vi "ImageInputToMatrix.vi"(0 "Path":path=path "U:/phys 434/Project/Suggested Images For Processing/OrlalaAndElana.JPG") -> (1 "Picture":picture, 6 "Image Data matrix":dbl[][](array[numeric]), 7 "image data":T2={"image type"=0, "image depth"=24, "image"=array[3686400 elements], "mask"=[], "colors"=[], "Rectangle"={"left"=0, "top"=0, "right"=1280, "bottom"=960}}, 8 "Image Data Vector":dbl[](array[numeric]))   [LabVIEW 2014]
uses:
  <vilib>/picture/picture.llb/imagedata.ctl
  <vilib>/Analysis/Matrix/Datatypes/RealMatrix.ctl
  <vilib>/Analysis/Matrix/Numeric/Conversions/Array To Matrix - RA2.vi
  <vilib>/Analysis/Matrix/NI_Matrix.lvlib
panel:
  out "Real Matrix":T1
  out "raw image data length":i32=3686400
  out "Image Data matrix size":i32[](array[numeric])=[1280, 960]
  out "Image Data Vector Size":i32=1228800
  out "raw image data":u8[](array[numeric])
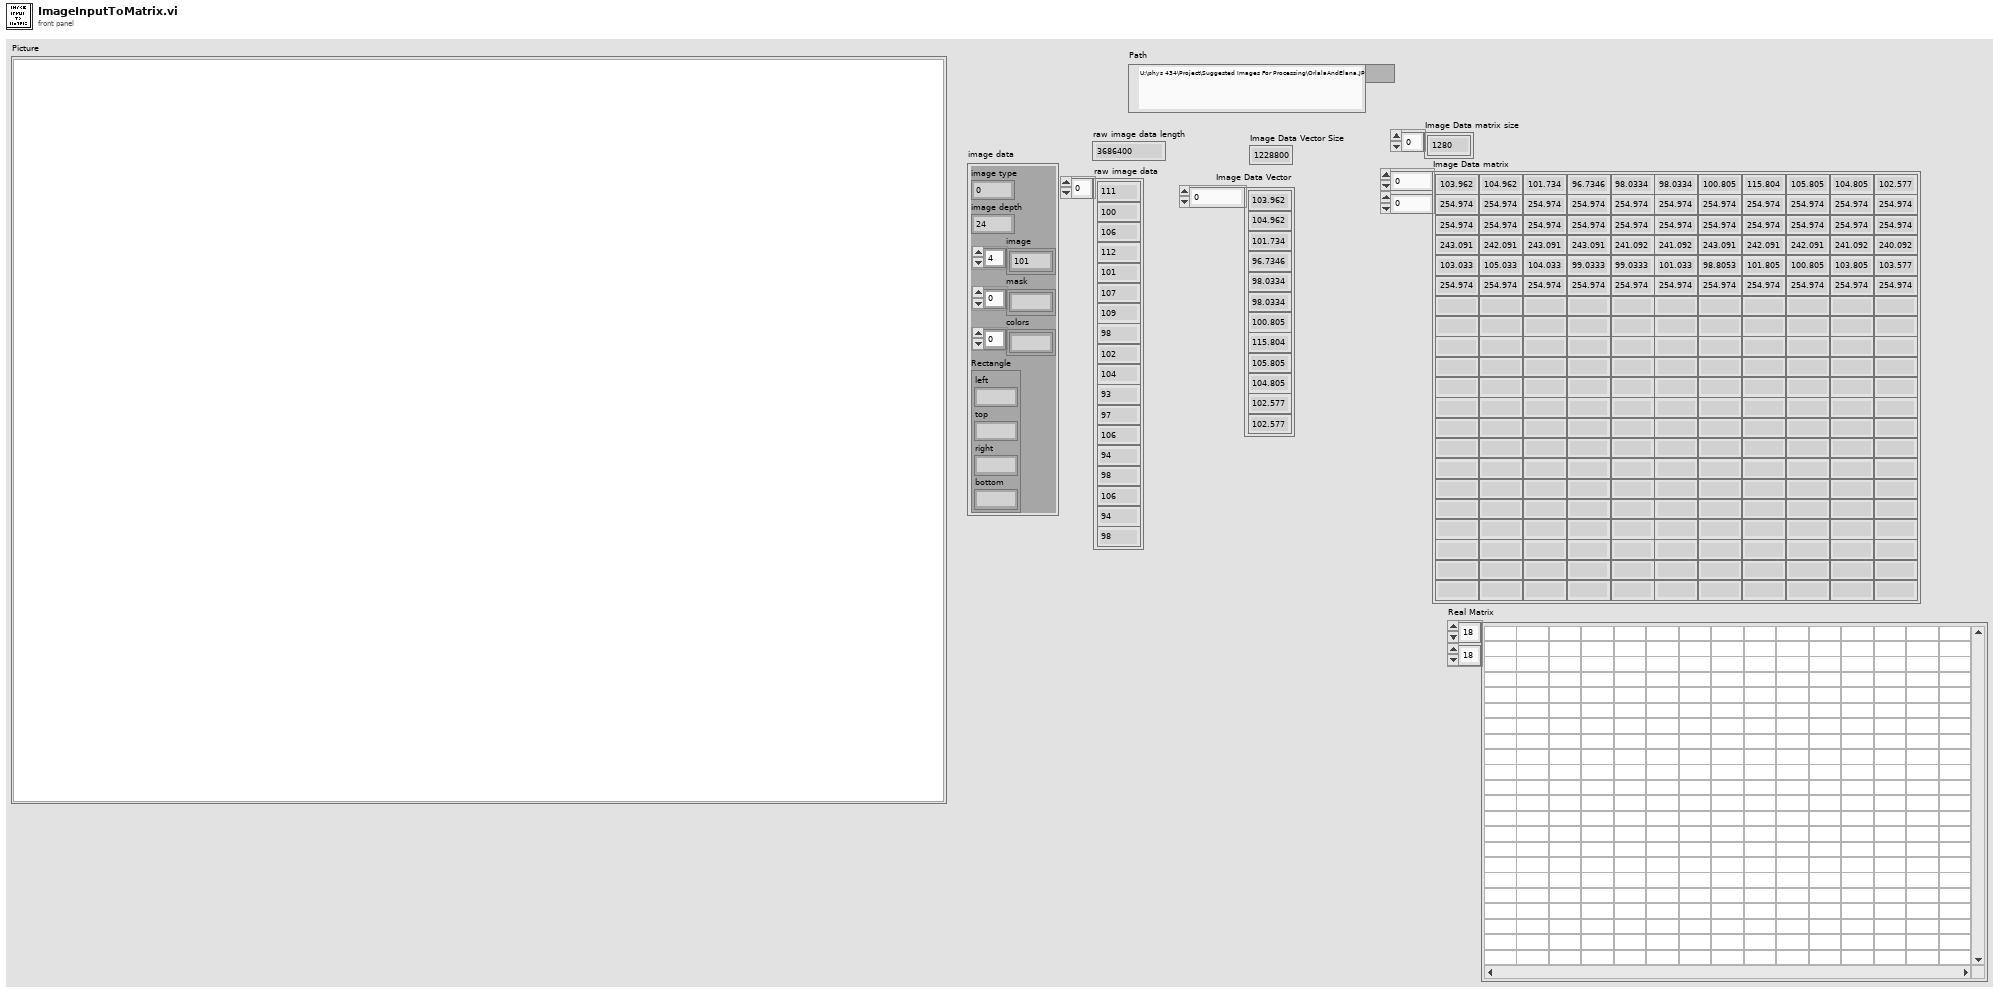
[diagram p1: front panel]
types:
  T1 = typedef "NI_Matrix.lvlib/RealMatrix.ctl" = dbl[][]
  T2 = typedef "imagedata.ctl" = cluster{"image type":i32, "image depth":i32, "image":u8[], "mask":u8[], "colors":u32[], "Rectangle":cluster{"left":i16, "top":i16, "right":i16, "bottom":i16}}
  T3 = cluster{"left":i16, "top":i16, "right":i16, "bottom":i16}
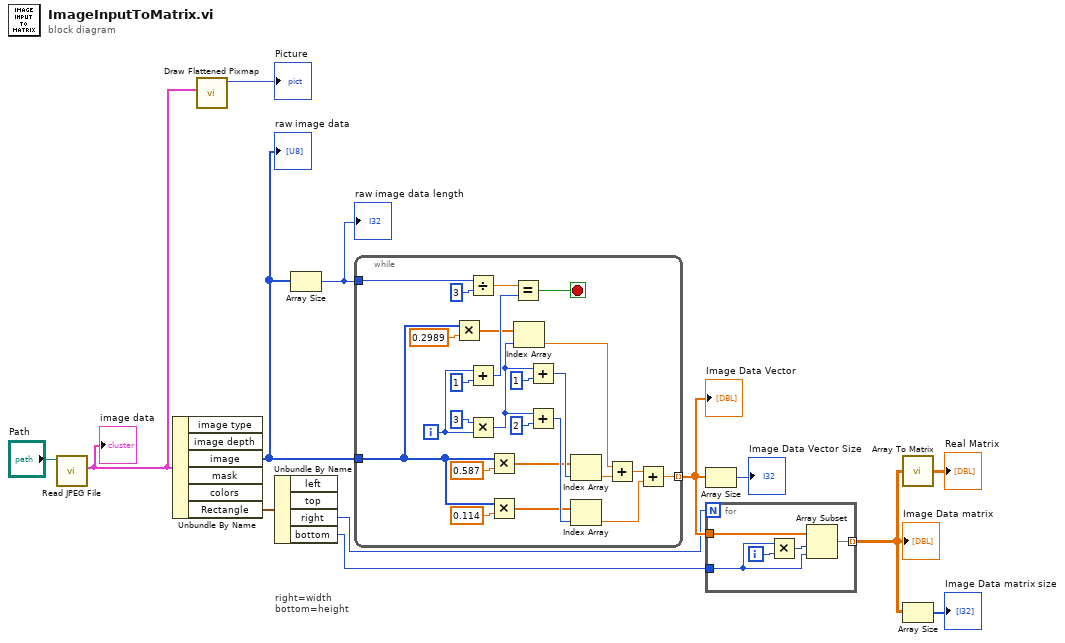
[diagram p0: block diagram]
diagram:
  # "right=width\nbottom=height"
  n1 = call <vilib>:"Read JPEG File.vi"("path to JPEG file"="Path") -> ("image data"=w2:T2)  [unwired: 8 in, 2 out]
  "image data" <- w2
  n2 = Unbundle By Name(w2) -> ("image"=w11:u8[], "Rectangle"=w12:T3)  [unwired: 4 out]
  "raw image data" <- w11
  n3 = call <vilib>:"Draw Flattened Pixmap.vi"("image data"=w2) -> ("new picture"=→"Picture":picture)  [unwired: 8 in]
  n4 = Unbundle By Name(w12) -> ("right"=w7:i16, "bottom"=w6:i16)  [unwired: 2 out]
  n5 = Array Size(array=w11) -> (size(s)=w5:i32)
  "raw image data length" <- w5
  n6 = while {
    tunnel: w11 -> [w15]
    tunnel: w5 -> [w31]
    tunnel: [w22] -> w8 mode=indexing
    i -> [w28]
    stop <- w29 stop-if-true
    n7 = Multiply(x=w15, y=0.2989) -> (x*y=w23:dbl[])
    n8 = Divide(x=w31, y=3) -> (x/y=w25:dbl)
    n9 = Add(x=w28, y=1) -> (x+y=w26:i32)
    n10 = Multiply(x=3, y=w28) -> (x*y=w36:i32)
    n11 = Multiply(x=w15, y=0.587) -> (x*y=w17:dbl[])
    n12 = Multiply(x=w15, y=0.114) -> (x*y=w16:dbl[])
    n13 = Equal?(x=w25, y=w26) -> (x = y?=w29:bool)
    n14 = Index Array(array=w23, index=w36) -> (element=w21:dbl)
    n15 = Add(x=w36, y=1) -> (x+y=w33:i32)
    n16 = Add(x=w36, y=2) -> (x+y=w32:i32)
    n17 = Index Array(array=w17, index=w33) -> (element=w20:dbl)
    n18 = Index Array(array=w16, index=w32) -> (element=w19:dbl)
    n19 = Add(x=w21, y=w20) -> (x+y=w38:dbl)
    n20 = Add(x=w38, y=w19) -> (x+y=w22:dbl)
  }
  "Image Data Vector" <- w8
  n21 = Array Size(array=w8) -> (size(s)=→"Image Data Vector Size":i32)
  n22 = for {
    N: w7 -> [_]
    tunnel: w6 -> [w41]
    tunnel: w8 -> [w40]
    tunnel: [w39] -> w4 mode=indexing
    i -> [w43]
    n23 = Multiply(x=w41, y=w43) -> (x*y=w42:i32)
    n24 = Array Subset(array=w40, index=w42, length=w41) -> (w39:dbl[])
  }
  "Image Data matrix" <- w4
  n25 = call-poly <vilib>:"Array To Matrix.vi"("Real 2D Array"=w4) -> ("Real Matrix"=→"Real Matrix":T1)
  n26 = Array Size(array=w4) -> (size(s)=→"Image Data matrix size":i32[])
